vi "neuKLEIN.vi"() -> ()   [LabVIEW 2016] (continued)
  in  "FPGA_DIO_Labels":T54={"Array"=["PB_0.20 - Image Freq Selector", "PB_0.12 - Blue Trap or Image Selector", "PB_0.22 - Blue Cold MOT TTL", "PB_0.17 - Blue Hot MOT Freq Selector", "***** BROKEN ***** BNC snapped, just needs to be replaced", "PB_0.19 - ODT Dimple (Sheet) Light Trigger", "PB_0.21 - ODT Loading Trap Light Trigger", "PB_1.00 - B field - Switch 0", "PB_1.07 - LCR Switch", "PB_1.10 - B field - Switch 1", "", "", "", "", "", "", "", "", "", "", " ", "", "", ""], "PB_0_Ch_Labels\n"=["0", "1", "2", "3", "4", "5", "6", "7", "8", "9", "10", "11", "12", "13", "14", "15", "16", "17", "18", "19", "20", "21", "22", "23", "24", "25", "26", "27", "28", "29", "30", "31"]}
  in  "FPGA_AO_Labels":T54={"Array"=["************BORKED************", "************BORKED************", "Blue MOT B-field gradient (external ADG419 switches to Red MOT gradient)", "6221 (ODT card) Waveform trigger", "X Trim Coil (Driving BioChip)", "Y Trim Coil", "Z Trim Coil", "LCR Setting", "Blue Laser Frequency Selector", "Blue MOT Power Setpoint", "", "", "", "", "", "", "", "", "", "", " ", "", "", ""], "PB_0_Ch_Labels\n"=["0", "1", "2", "3", "4", "5", "6", "7", "8", "9", "10", "11", "12", "13", "14", "15", "16", "17", "18", "19", "20", "21", "22", "23"]}
  in  "Update FPGA Ctrl":bool
  out "get_loop_time":u32
  out "error out":errorcluster={"status"=TRUE, "code"=-2145378293, "source"="Initboard.vi: Unknown or reserved error"}
  out "Handle Out":i16=16384
  out "Pico Scope Info":T55={"Driver Version"="1.1.4.20", "USB Version"="2.0", "Hardware"="1", "Variant"="5243B", "Batch and Serial"="CW334/117", "Cal Date"="20Mar14", "Kernel Version"="1.0", "Digital HW Version"="1", "Analogue HW Version"="1", "Firmware 1"="1.3.3.0", "Firmware 2"="1.0.24.0"}
  out "Control Reference Cluster":T56={"Controls[]"=[refnum, refnum, refnum, refnum, refnum, refnum, refnum, refnum, refnum, refnum, refnum, refnum, refnum, refnum, refnum, refnum, refnum, refnum, refnum, refnum, refnum, refnum, refnum, refnum, refnum, refnum, refnum, refnum, refnum, refnum, refnum, refnum, refnum, refnum, refnum, refnum, refnum, refnum, refnum, refnum, refnum, refnum, refnum, refnum, refnum, refnum, refnum, refnum, refnum, refnum, refnum, refnum, refnum, refnum, refnum, refnum, refnum, refnum, refnum, refnum, refnum, refnum, refnum, refnum, refnum, refnum, refnum, refnum, refnum, refnum, refnum, refnum, refnum, refnum, refnum, refnum, refnum, refnum, refnum, refnum, refnum, refnum, refnum, refnum, refnum, refnum], "Control Names"=["Control Tab Control", "Start Experiment", "Shutdown Experiment", "Exp Running", "Camera Ready", "Trigger Snap Mode", "Number", "Set Analysis Mode", "Temp. (K) - X", "Temp. (K) - Y", "Drop Time", "Scan Name", "Current Param. Values", "output cluster", "Take Pictures", "Abort Scan", "Scan Progress", "Information Tab Control", "Trap Frequencies", "Phase Space Density", "Break Loop", "Picoscope Ready", "Wavemeter", "Stat. Limits", "Num and Temp Stats", "Stats Flag", "cRIO Ready", "XML File Location", "Load", "XML Filename", "SaveButton", "current spinal_column MD5", "Agilent E3631A Settings", "Program Agilent", "PicoScope", "Intitialize PicoScope", "Novatech Synth Settings", "Synth Notes", "FPGA_panel_tab_ctrl", "6229 Green Lattice Inputs", "Green Lattice Waveform Graph", "ODT Params", "ODT Waveform Graph", "Red MOT 87 Inputs", "Red 87 Waveform Graph", "Red MOT 87 Notes", "Red MOT 88 Inputs", "Red 88 Waveform Graph", "Red MOT 88 Notes", "6713 Blue MOT", "Blue MOT Waveform Graph", "Blue MOT Trapping Notes", "PixelFly Status", "Buffer status", "PixelFly Controls", "Experimental Variables", "Calculated Experimental Values", "Scan Parameters", "48ch_pb_array", "PB_Labels_Tab", "error out", "Pico Scope Info", "Handle Out", "Control Reference Cluster", "Update FPGA Ctrl", "FPGA_AO_Labels", "FPGA_DIO_Labels", "get_loop_time", "GIANT Atoms", "Giant Data Cuts", "Pico Scope Channel A", "Pico Scope Channel B", "Atom Image", "Background Image", "Atoms - BG", "Atom Closeup", "OD", "Atom Number Chart", "Data Cuts", "Best Fit Parameter Cluster", "Elapsed time ( ms)", "Temperature Chart", "FPGA_Labels", "FPGA_cntrl", "pb_label_cluster 2", "pb_label_cluster"]}
  # "Select a PB Channel to set with a phase time for evaporation or whatever"
  # "Camera Controls"
  # "Camera Indicators"
  # "NOTE: 2015.10.19 - Jim\nDouble Shot is currently the only image mode supported.\nBackground subtraction will fail if the mode is changed"
  # "Status flags"
  # "Buffer errors"
  # "Memory usage"
  # "Center Freq. [MHz] (0)"
  # "Dither Amp. [kHz] (1)"
  # "Red Boson Power (2)"
  # "Red B-Field Gradient (3)"
  # "OUTPUT UNRELIABLE (4)"
  # "Image VCO Freq. (5)"
  # "Blue MOT VCO Freq. (6)"
  # "Spin Pol VCA (7)"
  # "Trap - Center Freq. (0)"
  # "Trap - Dither Amp. (1)"
  # "Trap - Power (2)"
  # "Z Trim [LO] (3)"
  # "Stir - Center Freq. (4)"
  # "Stir - Dither Amp. (5)"
  # "Stir - Power (6)"
  # "Z Trim [HI] (7)"
  # "Notes below cluster describe the variables used for each formula and \neach variable has a designation of SET or CALC as explained here\n\nSET - user defined, defines the output waveform \nCALC - program calculated value that will be updated in the entry field, input is ignored"
  # "Difference between \"Evaporation Formula\" and \"Evap - Calc Tau\" is mostly in defining\nthe endpoint of the trajectory. By calculating tau you can specify the final voltage of\nthe waveform."
  # "Power Law\ny = const + (init - const)* t^eta\n\nConstant - SET - constant offset\nInitial Value - SET - starting point for ramp\nFinal Value - CALC - final value of waveform at the end of the phase\nTau - CALC - forced to zero (not used for power law)\nEta - SET - power law dependence on time, positive (neg causes error)"
  # "Evaporation Formula\ny = const +  (init - const) / (1 + t/tau)^beta\nbeta is a function of eta as defined in PRA 64, 051403 \n\nConstant - SET - constant offset\nInitial Value - SET - starting point for ramp\nFinal Value - CALC - final value of waveform at the end of the phase\nTau - SET - time constant for the evaporation\nEta - SET - ratio of temperature over trap depth"
  # "Evap - Calc Tau\ny =  init / (1 + t/tau)^beta\ntau =  tf * (1 / ( 1 - ( final / init ))**(1 / beta) - 1)\ntf is the final time (total phase time)\nbeta is a function of eta\n\nConstant - CALC - forced to zero (not used)\nInitial Value - SET - starting point for ramp\nFinal Value - SET - final value of waveform at the end of the phase\nTau - CALC - time constant for the evaporation\nEta - SET - ratio of temperature over trap depth"
  # "Notes below  describe the variables used for each formula and each variable has a designation of SET or NA as explained here\n\nSET - user defined, defines the output waveform \nNA - input in this field is ignored for this function\n\nConversion selection is currently disabled (2018.11.01) can be enabled by modifying the Arb Waveform subvi to include calc"
  # "Evap - Calc Tau\ny =  init / (1 + t/tau)^beta\ntau =  tf * (1 / ( 1 - ( final / init ))**(1 / beta) - 1)\ntf is the final time (total phase time)\nbeta is a function of eta\n\nConstant - CALC - forced to zero (not used)\nInitial Value - SET - starting point for ramp\nFinal Value - SET - final value of waveform at \n                                 the end of the phase\nTau - CALC - time constant for the evaporation\nEta - SET - ratio of temperature over trap depth"
  # "Power Law\ny = const + (init - const)* t^eta\n\nConstant - SET - constant offset\nInitial Value - SET - starting point for ramp\nFinal Value - SET - final value of waveform at the end of the phase\nTau - CALC - forced to zero (not used for power law)\nEta - SET - power law dependence on time, positive (neg causes error)"
  # "Exponential\ny = (vo-constant) * exp(t/(tau)) + constant;\ntau = time / ln(vf/(vo-constant)); (time is the total phase time)\n\nConstant - SET - constant offset\nInitial Value - SET - starting point for ramp\nFinal Value - SET - final value of waveform at the end of the phase)\nDegree - NA"
  # "Evaporation Formula\ny = const +  (init - const) / (1 + t/tau)^beta\nbeta is a function of eta as defined in PRA 64, 051403 \n\nConstant - SET - constant offset\nInitial Value - SET - starting point for ramp\nFinal Value - CALC - final value of waveform at \n                                     the end of the phase\nTau - SET - time constant for the evaporation\nEta - SET - ratio of temperature over trap depth"
  # "Constant\ny = Constant + Initial + Final; \n\nConstant - SET - can still be used for conversions - constant offset\nInitial Value - SET - starting point for ramp\nFinal Value - SET\nDegree - NA"
  # "Tanh\ny = (vf - vo)/2*(tanh(slope*2*pi*t - slope*pi) +1) + vo; \n\nConstant - NA - can still be used for conversions - constant offset\nInitial Value - SET - starting point for ramp\nFinal Value - SET - Final value of the ramp\nDegree - SET - sets the slope of the Tanh (bigger is steeper)"
  # "Difference between \"Evaporation Formula\" and \"Evap - Calc Tau\" is mostly in defining\nthe endpoint of the trajectory. By calculating tau you can specify the final voltage of\nthe waveform."
  # "(0) Arm A"
  # "(1) Arm B"
  # "(2) Arm C"
  # "(3) Unused"
  # "(0) Arm A"
  # "(1) Arm B"
  # "(2) Arm C"
  # "(3) Unused"
  # "Constant Operation Control"
  # "Boolean Operation Control"
  # "Custom Operation Controls"
  # "Constant Operation Control"
  # "Boolean Operation Control"
  # "Custom Operation Controls"
  # "Constant Operation Control"
  # "Boolean Operation Control"
  # "Custom Operation Controls"
  # "Constant Operation Control"
  # "Boolean Operation Control"
  # "Custom Operation Controls"
  # "Constant Operation Control"
  # "Boolean Operation Control"
  # "Custom Operation Controls"
  # "Constant Operation Control"
  # "Boolean Operation Control"
  # "Custom Operation Controls"
  # "Constant Operation Control"
  # "Boolean Operation Control"
  # "Custom Operation Controls"
  # "Constant Operation Control"
  # "Boolean Operation Control"
  # "Custom Operation Controls"
  # "Constant Operation Control"
  # "Boolean Operation Control"
  # "Custom Operation Controls"
  # "Constant Operation Control"
  # "Boolean Operation Control"
  # "Custom Operation Controls"
  # "Constant Operation Control"
  # "Boolean Operation Control"
  # "Custom Operation Controls"
  # "Constant Operation Control"
  # "Boolean Operation Control"
  # "Custom Operation Controls"
  # "Constant Operation Control"
  # "Boolean Operation Control"
  # "Custom Operation Controls"
  # "Constant Operation Control"
  # "Boolean Operation Control"
  # "Custom Operation Controls"
  # "Constant Operation Control"
  # "Boolean Operation Control"
  # "Custom Operation Controls"
  # "Constant Operation Control"
  # "Boolean Operation Control"
  # "Custom Operation Controls"
  # "Synth Layout\n---------------------\nSyn. 0   |   Syn. 1   | \n-------- |---------- |\nSyn. 2   |   Syn. 3   |\n\n*2D grid is collapsed to 1D so be careful with addressing if adding more synths"
  # "Things to do for Pico VI\n2017.09.11 \n- Make this control more versatile, not only having the conversions work at 15bit resolution and the threshold needs to work for any range setting\n- Auto trigger time should have option to set time to wait as some factor of the total experimental time (like 1.2*(total PB time)"
  # "2016.12.12 - Currently back-end cnoversion assume the scope is in 15bit mode with the range at 5V."
  # "2018.10.31\nNOTE: (JAA) This triggerable functionality of the Agilent has been abandoned. It kind of works but is not reliable. The code should be taken out of the program entirely and only the single-use programmable piece should be kept (the part activated by pressing Program Agilent) as this is the reliable bit of code."
  # "Since the Agilent is slow to communicate the program will skip programming if the \"Auto Program Agilent\" switch is disabled.  If \"Auto Program\" is enabled the settings to the far left are used to program the Agilent.\n\nAdditionally, the Agilent has an internal software trigger that can a single channel between two current setpoints. The clock is not referenced to the Pulseblaster so be careful with timing when using the Triggered Agilent Settings. To enabled this mode use the \"Agilent Software Trigger\" swithc.\n\nUse the \"Program Agilent\" button to perform a one-time write (with settings on the far left) to avoid having the slow response of the supply during data scans.\n\nNOTE: When setting only current values the program will default to setting the maximum allowed voltage for a given channel."
  # "6V (2017.06.15)\n\nReported Current = \nSet Cur - 0.003A\n\nActual Current = \nSet Cur - 0.0015A"
  # "+25V (2017.06.15)\n\nReported Current = \nSet Cur + 0.002A\n\nActual Current = \nSet Cur + 0.002A"
  # "-25V (2017.06.15)\n\nReported Current = \nSet Cur\n\nActual Current = \nSet Cur"
  # "Beware of the offset in set, reported and actual current from Agilent channels. Below are corrections measured for each channel"
  # "--25V  Measurements"
  # "+25V  Measurements"
  # "6V  Measurements"
  # "-25V Output Settings"
  # "+25V Output Settings"
  # "6V Output Settings"
  # "When saving and loading the .dat file for experiments, you must ensure that the type definition is consistent between the version of spinal_column you are attempting to use. (i.e. the saved data type def and the current version type def must be exactly the same)\n\nThe MD5 hash is a unique string for the current status of the spinal column type defintiion. This MD5 will be saved into the filename for the dat files and checked when loading files."
  # "Click to save an xml file of the current experimental parameters\nto the raw_data folder indicated in the \"scan parameters\" tab"
  # "of"
  # "<-- Pump Side"
  # "Source Side -->"
  # "Digital Input Labels"
  # "IMPORTANT INFO:\n\n- For explanations of the available operations please refer to the \"FPGA operations.pdf\" file included in the neuKLEIN project.\n(In manual describe how you have to deploy the library to the RT target. Really need to get references for learning)\n\n- When using the scan functionality to take data, Channel to change will identify the channel while Phase to change will only be used for the \"Custom operation\" where it identifies which Output Value to change. The constant & Boolean operations have separate cases for controllnig these outputs.\n\n- BOP protection causes jumps greater than 1.5A to be ramped at a rate of 100A/s (or 100mA/ms). When the current gets within 1.5A the control voltage will jump the BOP to the final setpoint."
  # "Analog Output Labels"
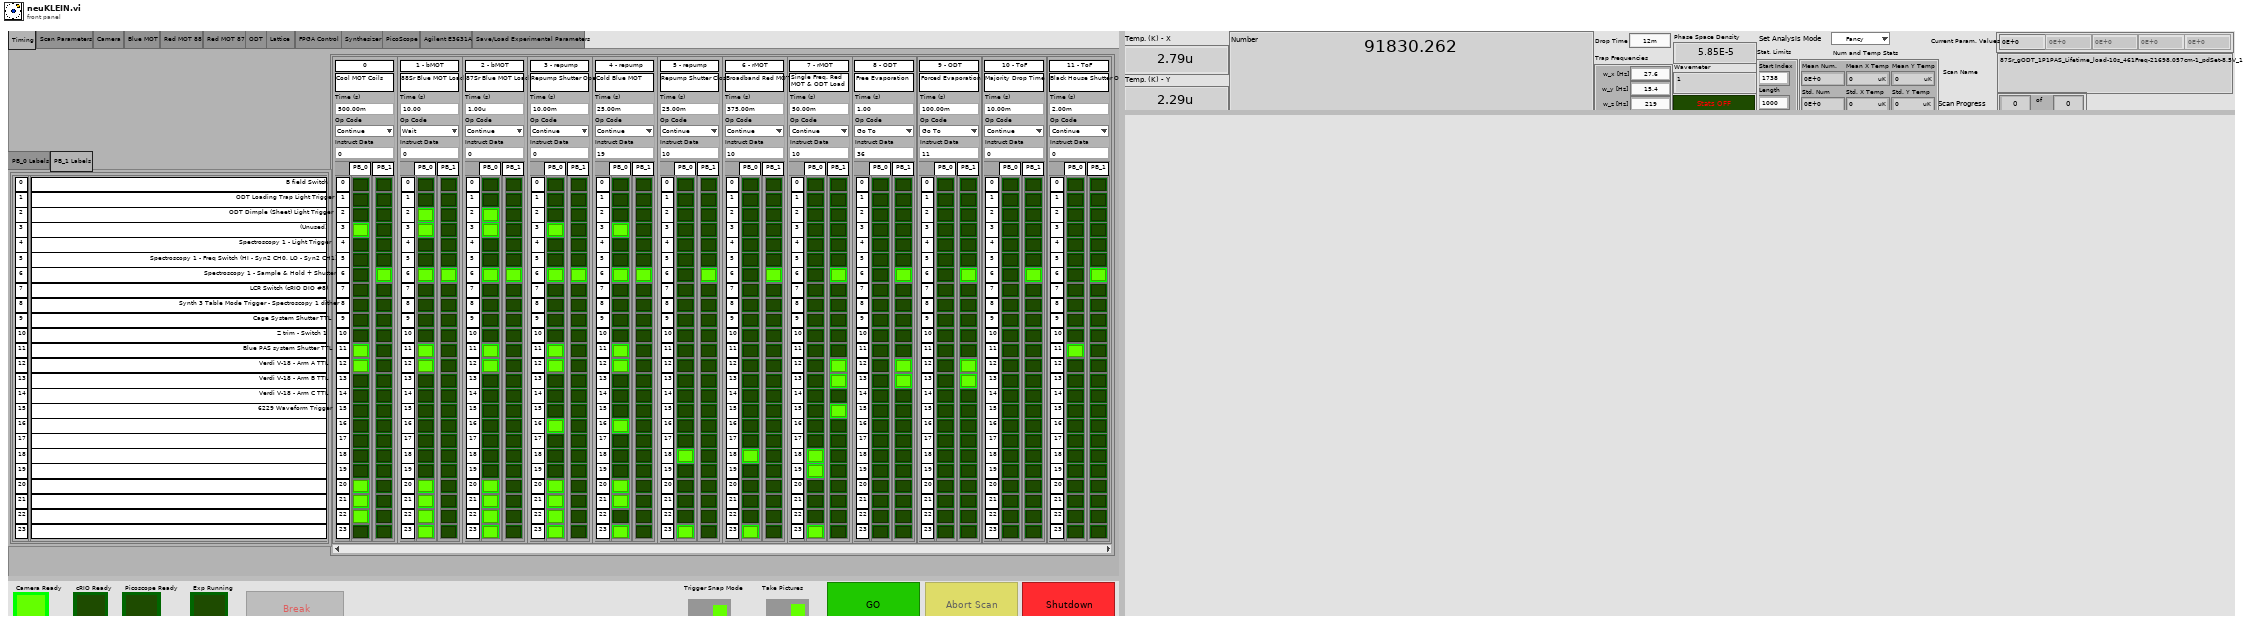
[diagram p1: front panel]
types:
  T1 = enum32{"Timing", "Scan Parameters", "Camera", "Blue MOT", "Red MOT 88", "Red MOT 87", "ODT", "Lattice", "FPGA Control", "Synthesizer", "PicoScope", "Agilent E3631A", "Save/Load Experimental Parameters"}
  T2 = typedef "pb_labels_v2.ctl" = cluster{"Array":string[], "PB_0_Ch_Labels\n":string[]}
  T3 = typedef "48ch_pb_array.ctl" = T4[]
  T4 = typedef "48ch_single_timing_column_condensed.ctl" = cluster{"Label and Instructions":cluster{"Column Number":string, "Comments":string, "Time (s)        ":dbl, "Op Code":i32, "Instruct Data":i32}, "PB_1_Bools":bool[], "Column Number":string, "Column Number 2":string, "PB_0_Bools":bool[], "Ch_Labels":string[]}
  T5 = typedef "ScanParametersPanel.ctl" = cluster{"Initial Values":dbl[], "Final Values":dbl[], "Step Sizes":dbl[], "Parameters to Change":T6[], "Channels to Change":u32[], "Number of Parameters to Scan":i32, "Parameter Nickname (no spaces)":string[], "Scan Base Name":string, "Raw_Data Folder":path, "ROI Parameters":T7, "Drop Time (ms)":dbl, "Phases To Change":u32[], "Scan Pulseblaster Channel With Parameter":T8, "Preserve Waveform\nContinuity":bool, "Generated Array Type":enum16{"Custom Array From File", "Default (old way)"}, "Master Batch Third Column":dbl, "Master Batch Fourth Column":dbl, "Master Batch Fifth Column":dbl, "Current Param. Values":dbl[]}
  T6 = typedef "ParameterToChange.ctl" = enum16{"Dummy Variable", "Synth Amplitude", "Synth Frequency", "Synth Phase", "ODT Params Phase Time", "ODT Params Tau", "ODT Params Final Voltage", "ODT Params Initial Voltage", "ODT Params Eta", "Red Mot 88 Phase Time", "Red Mot 87 Phase Time", "Red Mot 88 Final Voltage", "Red Mot 88 Initial Voltage", "Red Mot 87 Final Voltage", "Red Mot 87 Initial Voltage", "PulseBlaster", "6713 Voltage", "Green Lattice Phase Time", "Green Lattice Initial Voltage", "Green Lattice Final Voltage", "Agilent Current Setpoint", "FPGA - Constant Op - Set", "FPGA - Bool Op - Output HI", "FPGA - Bool Op - Output LO", "FPGA - Custom Op"}
  T7 = typedef "ROI_set.ctl" = cluster{"Background Radius":dbl, "Atom Radius":dbl, "X Center":dbl, "Y Center":dbl}
  T8 = typedef "ScanPBandParam.ctl" = cluster{"Change PB Time Toggle":bool, "PB Channel":dbl, "Parameter Number":dbl}
  T9 = typedef "experimentalvariables.ctl" = cluster{"Pixel Size before binning (µm)":dbl, "Imaging Wavelength (m)":dbl, "Isotope":i32, "1P1 Linewidth (MHz)":dbl, "Imaging Detuning (MHz)":dbl, "Software Bin Size":u16, "Exp. Trigger ON time (ms)":dbl, "Path to spinapi.dll":path, "PB clock_freq (MHz)":dbl}
  T10 = cluster{"Absorption Cross Section (µm)":dbl, "Effective Pixel Area (µm^2)":dbl, "Effective Pixel Size (µm)":dbl}
  T11 = typedef "PixelFly_Control.ctl" = cluster{"Acquitsition Settings":T12, "Initialization":cluster{"Exposure mode":u16, "exp time":i32, "exp level":i32, "gain":i32, "boardid in":i32, "offset":i32, "V bin":i32, "H bin":i32, "trigger":bool, "Bit depth":T13}}
  T12 = typedef "Acquisition Settings.ctl" = cluster{"Buffer number":i32, "Size (Bytes)":i32, "initialized array":u16[][], "X Bin":i32, "Y Bin":i32, "Board Handle":u32, "Picture parameters":cluster{"ccdxsize":i32, "ccdy":i32, "pictx":i32, "picty":i32, "bitspixel":i32}, "Buffer Out":u16[]}
  T13 = typedef "Bit_Depth_Enum.ctl" = i32
  T14 = typedef "PixelFly Buffer Status.ctl" = cluster{"Write":bool, "Write done":bool, "Queued":bool, "Cancelled":bool, "Select":bool, "Select done":bool, "Burst":bool, "Size":bool, "Event":bool, "Timeout":bool, "Open":i32, "Map":i32, "Exposure":i32[], "Offset":i32[], "Size":i32[], "Transfer":i32[], "Total Size":i32}
  T15 = typedef "PixelFly Status Indicator.ctl" = cluster{"Board Parameters":cluster{"Type":u32, "Number":u32, "Initialized":bool, "Running":bool, "Lost head":bool, "CCD X size":u32, "CCD Y size":u32, "Mode":u32, "Exposure time":u32, "Exposure level":u32, "Horizontal bin":u32, "Vertical bin":u32, "Reg W":bool, "Gain":u32, "Pixel depth":i32, "Bit Shift":u32, "Offset":u32, "Last exposure":u32, "Double ":bool, "Light meter":bool, "Color":bool, "Open count":u32, "Active buffer":bool, "Next Buffer":bool}, "CCD temp":i32}
  T16 = typedef "6713_waveform_generation.ctl" = cluster{"Active Device":string, "Active Channels":bool[], "Waveform Parameters":T17, "Active Phases":bool[], "Phase Times":dbl[], "Trigger Channel":tag, "FIFO Buffer Size":dbl, "6713_ch_labels":T20}
  T17 = typedef "6713_waveform_parameter_array.ctl" = T18[][]
  T18 = typedef "6713_static_waveform_item.ctl" = cluster{"Constant":dbl, "Nickname":string, "Conversion":T19}
  T19 = typedef "Neutral_voltage_conversion_control.ctl" = enum16{"Volts", "B Field Grad (G/cm)", "Red Boson Cntr Freq (MHz)", "Red Boson Dither Amp (kHz)", "Red Boson Power (mW)", "Red 87 Trap Cntr Freq (MHz)", "Red 87 Trap Dither Amp (kHz)", "Red 87 Trap Power (mW)", "Red 87 Stir Cntr Freq (MHz)", "Red 87 Stir Dither Amp (kHz)", "Red 87 Stir Power (mW)", "ODT Sheet Trap Power (W)", "ODT Loading Trap Power (W)"}
  T20 = typedef "6713_ch_labels.ctl" = cluster{"Array":string[], "PB_0_Ch_Labels\n":string[]}
  T21 = typedef "6733_control_panel.ctl" = cluster{"Active Device":string, "Active Channels":bool[], "Waveform Parameters":T22, "Active Phases":bool[], "Phase Times":dbl[], "Trigger Channel":T24}
  T22 = typedef "6733_waveform_parameter_array.ctl" = T23[][]
  T23 = typedef "6733_waveform_item.ctl" = cluster{"Function":enum16{"Polynomial", "Exponential", "Constant", "Tanh"}, "Initial":dbl, "Final":dbl, "Degree":dbl, "Nickname":string, "Conversion":T19, "Constant":dbl}
  T24 = typedef "Trigger_Channel_Selector.ctl" = tag
  T25 = typedef "6221_panel.ctl" = cluster{"Waveform Parameters":T26, "Active Phases":bool[], "Active Channels":bool[], "Phase Times (s)":dbl[], "Active Device":string, "Trigger Channel":tag, "Evaporation Phase":dbl, "Evaporation Channel":dbl}
  T26 = typedef "6221_waveform_input.ctl" = T27[][]
  T27 = typedef "6221_waveform_param.ctl" = cluster{"Initial Value":dbl, "Final Value":dbl, "Tau":dbl, "Eta":dbl, "Nickname":string, "Function Type":enum16{"Constant", "Power Law", "Evap - Calc Tau", "Evaporation Formula", "Tanh", "Exponential"}, "Conversion":T19, "Constant":dbl}
  T28 = typedef "6229_arb_waveform_generation.ctl" = cluster{"Active Device":string, "Active Channels":bool[], "Active Phases":bool[], "Phase Times":dbl[], "Trigger Channel":tag, "FIFO Buffer Size":dbl, "Sample Step Time (us)":dbl, "Initialization Parameters":cluster{"Enable Initialization":bool, "Initial Values":dbl[]}, "Waveform Parameters":T29}
  T29 = typedef "6229_evap_waveform_input.ctl" = T27[][]
  T30 = typedef "op_ctrl_cluster.ctl" = cluster{"Channel 0":T31, "Channel 1":T31, "Channel 2":T31, "Channel 3":T31, "Channel 4":T31, "Channel 5":T31, "Channel 6":T31, "Channel 7":T31, "Channel 8":T31, "Channel 9":T31, "Channel 10":T31, "Channel 11":T31, "Channel 12":T31, "Channel 13":T31, "Channel 14":T31, "Channel 15":T31}
  T31 = typedef "op_ctrl_element.ctl" = cluster{"Operation":i16, "Input A":T32, "Output - LO":T33, "Output - HI":T33, "Inputs":T32[], "Output Values":T33[], "Num. Inputs":i32, "Set Point":T33, "Inv.":bool[], "Inv. A":bool, "Inv. B":bool, "Input B":T32}
  T32 = typedef "DIO_selector.ctl" = i32
  T33 = typedef "output_value.ctl" = fxp<+/-,20,5>
  T34 = typedef "op_label_cluster.ctl" = cluster{"Channel 0":T35, "Channel 1":T35, "Channel 2":T35, "Channel 3":T35, "Channel 4":T35, "Channel 6":T35, "Channel 5":T35, "Channel 7":T35, "Channel 8":T35, "Channel 9":T35, "Channel 10":T35, "Channel 11":T35, "Channel 12":T35, "Channel 13":T35, "Channel 14":T35, "Channel 15":T35}
  T35 = typedef "op_label_element.ctl" = cluster{"Channel Description":string}
  T36 = typedef "Synth_controls.ctl" = cluster{"Channel Settings":T37[], "Active Chans":bool[], "COM Port":refnum<visa-resource-name>, "Table Mode":T38}
  T37 = typedef "synth_channel.ctl" = cluster{"Voltage (Amp.) ":dbl, "Frequency (MHz)":dbl, "Phase (deg)":dbl, "Nickname":string}
  T38 = typedef "table_mode.ctl" = cluster{"Initial Freq.(MHz)":dbl, "FinalFreq":dbl, "Freq. Step (MHz)":dbl, "Voltage (Amp.)":dbl, "Asc. & Desc.":bool, "Custom Frequencies":dbl[], "Custom Amplitude":dbl[], "Table Mode Switch":bool, "Array Gen":enum16{"Auto", "Custom"}, "Randomize":bool, "Continuous":bool}
  T39 = typedef "pico_control_panel.ctl" = cluster{"Channel A Settings":T40, "Channel B Settings":T40, "Trigger Options":T41, "Pico Scope Inititalization Settings":T42, "Use PicoScope?":bool, "Acquisition Settings":cluster{"Pre Trigger Time (s)":dbl, "Post Trigger Time (s)":dbl, "Resolution (s)":dbl, "Four Channel Device":bool, "Number of Captures":dbl}}
  T40 = typedef "pico_channel_settings.ctl" = cluster{"Enabled":bool, "Coupling":i16, "Range":u16, "Analogue Offset":sgl}
  T41 = typedef "pico_trigger.ctl" = cluster{"Trigger Enabled":bool, "Trigger Source":enum16{"Channel A", "Channel B", "Channel C", "Channel D", "Ext."}, "Trigger Threshold (-5 to 5 V)":dbl, "Trigger Slope":u16, "Trigger Delay (s)":dbl, "Auto Trigger Time (ms)":i16}
  T42 = typedef "pico_init_settings.ctl" = cluster{"USB Power":bool, "Use Serial Number":bool, "Resolution":i32, "Serial Number":string, "Handle":i16}
  T43 = typedef "Settings_Control.ctl" = cluster{"VISA resource name":refnum<visa-resource-name>, "Voltage Set (6V max)":dbl, "Current Set (5A max)":dbl, "Voltage Set (25V max)":dbl, "Current Set (1A max)":dbl, "Voltage Set (-25V max)":dbl, "Current Set (1A max)":dbl, "6V Switch":bool, "+25V Switch":bool, "-25V Switch":bool, "Agilent E3631A Measurements":T44, "Triggered Agilent Settings":T45, "Auto Program Agilent":bool, "Agilent Software Trigger":bool}
  T44 = typedef "Measurement_Indicator.ctl" = cluster{"6V Actual Voltage Level (V)":dbl, "6V Actual Current Level (A)":dbl, "25V Actual Voltage Level (V)":dbl, "25V Actual Current Level (A)":dbl, "-25V Actual Current Level (A)":dbl, "-25V Actual Voltage Level (V)":dbl}
  T45 = typedef "Trigger_Settings.ctl" = cluster{"Trigger \nDelay (s)":dbl, "Enable +6V Channel":bool, "+6V Current":dbl, "Enable -25V Channel":bool, "-25V Current":dbl, "Enable +25V Channel":bool, "+25V Current":dbl}
  T46 = typedef "output_cluster.ctl" = cluster{"Number":dbl, "OD":dbl[][], "Data Cuts":dbl[][], "Temperature (K) x":dbl, "Temperature (K) y":dbl}
  T47 = typedef "numAndTempStats.ctl" = cluster{"Mean Num.":dbl, "Std. Num":dbl, "Mean X Temp":dbl, "Std. X Temp":dbl, "Mean Y Temp":dbl, "Std. Y Temp":dbl}
  T48 = cluster{"w_x [Hz]":dbl, "w_y [Hz]":dbl, "w_z [Hz]":dbl}
  T49 = typedef "Progress_Indicator.ctl" = cluster{"Current Pnt Num":i32, "Total Num Pts":i32}
  T50 = enum32{"Standard Image Information", "Picoscope traces", "Large OD Image", "cRIO Information", "Error Information"}
  T51 = cluster{"Temperature (K) x":dbl, "Temperature (K) y":dbl}
  T52 = typedef "Fit Parameter Cluster.ctl" = cluster{"Amplitude (OD)":dbl, "X Center (px)":dbl, "Y Center (px)":dbl, " X Width (um)":dbl, "Y Width (um)":dbl, "Aspect Ratio":dbl, "Rot. Angle (deg)":dbl}
  T53 = cluster{"Channel A Out":dbl[], "Channel A Out":dbl[]}[]
  T54 = typedef "portAssign_labels.ctl" = cluster{"Array":string[], "PB_0_Ch_Labels\n":string[]}
  T55 = cluster{"Driver Version":string, "USB Version":string, "Hardware":string, "Variant":string, "Batch and Serial":string, "Cal Date":string, "Kernel Version":string, "Digital HW Version":string, "Analogue HW Version":string, "Firmware 1":string, "Firmware 2":string}
  T56 = cluster{"Controls[]":refnum<vi>[], "Control Names":string[]}
  T57 = typedef "rydberg_state_machine_states.ctl" = enum16{"Initialize", "Idle", "Experiment Running", "Trigger Snap Mode", "Scan Mode", "Load Experiment", "Shutdown"}
  T58 = enum8{"Enabled", "Disabled", "Disabled and Grayed Out"}
  T59 = cluster{"Experimental Variables":T9, "Red MOT 88 Inputs":T21, "6713 Blue MOT":T16, "48ch_pb_array":T3, "Red MOT 87 Inputs":T21, "ODT Params":T25, "Agilent E3631A Settings":T43, "PixelFly Controls":T11, "Scan Parameters":T5, "PicoScope":T39, "6229 Green Lattice Inputs":T28, "Novatech Synth Settings":T36[][], "Control Reference Cluster":cluster{"Controls[]":refnum<vi>[], "Control Names":string[]}, "FPGA_cntrl":T30}
  T60 = cluster{"Initial Values":refnum<vi>, "Final Values":refnum<vi>, "Step Sizes":refnum<vi>}
  T61 = cluster{"Channels to Change":refnum<vi>, "Phases To Change":refnum<vi>}
  T62 = typedef "DialogType.ctl" = u16
  T63 = typedef "spinal_column.ctl" = cluster{"Experimental Variables":T9, "Red MOT 88 Inputs":T21, "6713 Blue MOT":T16, "48ch_pb_array":T3, "Red MOT 87 Inputs":T21, "ODT Params":T25, "Agilent E3631A Settings":T43, "PixelFly Controls":T11, "Scan Parameters":T5, "PicoScope":T39, "6229 Green Lattice Inputs":T28, "Novatech Synth Settings":T36[][], "Control Reference Cluster":cluster{"Controls[]":refnum<vi>[], "Control Names":string[]}, "FPGA_cntrl":T30}
  T64 = typedef "LVCursorListTypeDef.ctl" = cluster{"Name":string, "Color":u32, "Style":u8, "Point Style":u8, "Name Visible":bool, "Allow Drag":bool, "Cursor Mode":u32, "Plot":i32, "Index":i32, "Position":cluster{"X":dbl, "Y":dbl}, "X Scale":u32, "Y Scale":u32, "Watch Plots":i32[], "Watch All Plots":bool, "Plot Area":i32, "Label Offset":cluster{"X":dbl, "Y":dbl}}[]
  T65 = cluster{"Temperature (K) x":dbl, "Temperature (K) y":dbl}[]
  T66 = cluster{"XScale.Maximum":dbl, "History Data":dbl[], "History Data":cluster{"Temperature (K) x":dbl, "Temperature (K) y":dbl}[]}
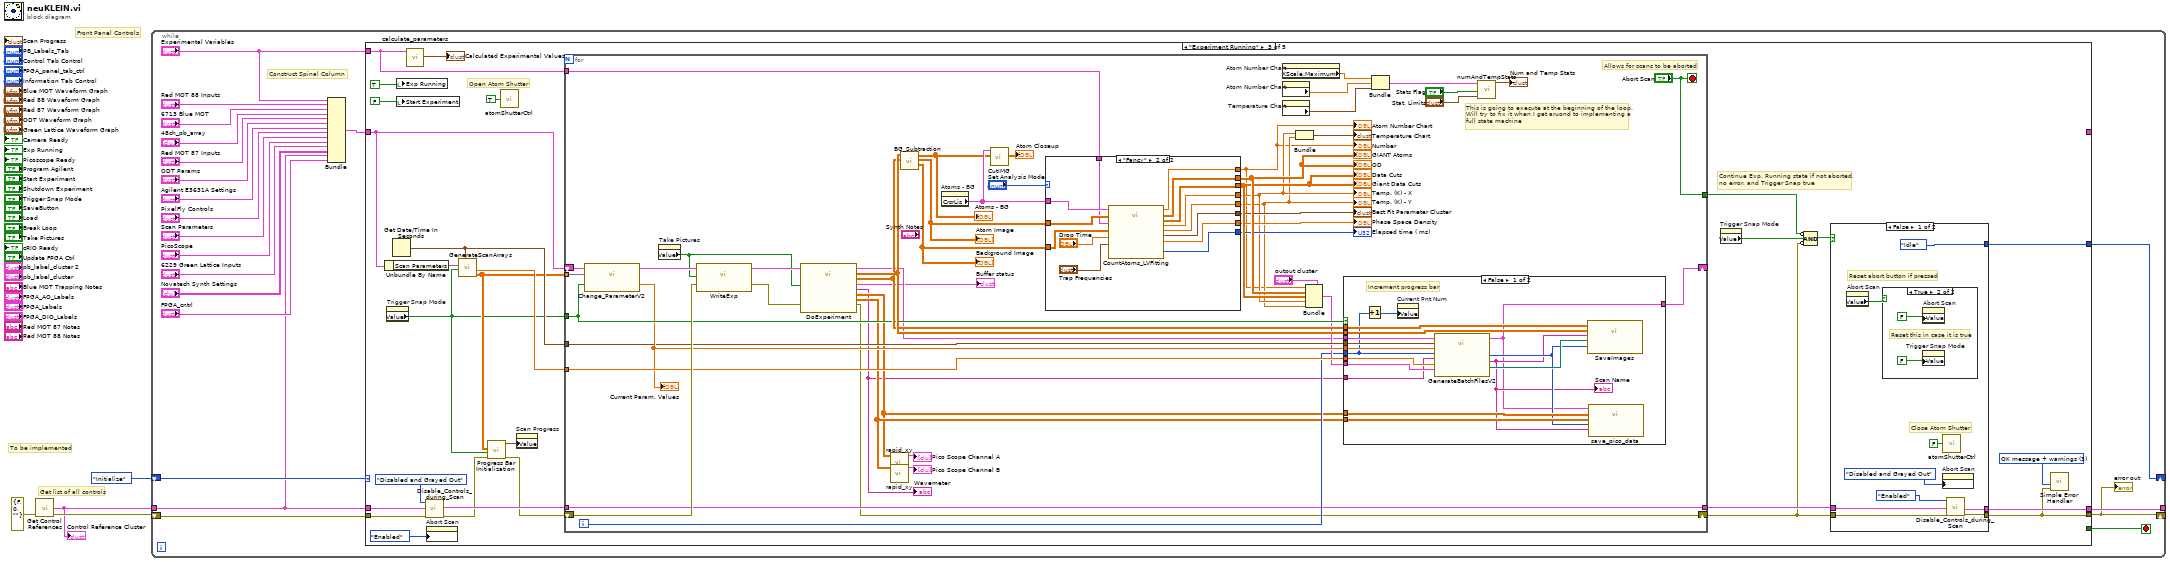
[diagram p0: block diagram]
diagram:
  # "To be implemented"
  # "Get list of all controls"
  # "Front Panel Controls"
  n1 = call "Get Control References.vi"("error in"=errorcluster {"status"=FALSE, "code"=0, "source"=""} ("error constant")) -> ("error out"=w2:errorcluster, "Control Reference Cluster"=w1:T56)  [unwired: 3 in]
  "Control Reference Cluster" <- w1
  n2 = while {
    shift-right: [w23] -> _
    shift-left: rydberg_state_machine_states."Initialize" -> [w25]
    shift-right: [w7] -> _
    shift-left: w2 -> [w24]
    tunnel: w1 -> [w5]
    tunnel: [w12] -> _
    stop <- w22 stop-if-true
    # "Construct Spinal Column"
    n3 = Bundle("Experimental Variables"="Experimental Variables", "Red MOT 88 Inputs"="Red MOT 88 Inputs", "6713 Blue MOT"="6713 Blue MOT", "48ch_pb_array"="48ch_pb_array", "Red MOT 87 Inputs"="Red MOT 87 Inputs", "ODT Params"="ODT Params", "Agilent E3631A Settings"="Agilent E3631A Settings", "PixelFly Controls"="PixelFly Controls", "Scan Parameters"="Scan Parameters", "PicoScope"="PicoScope", "6229 Green Lattice Inputs"="6229 Green Lattice Inputs", "Novatech Synth Settings"="Novatech Synth Settings", "Control Reference Cluster"=w5, "FPGA_cntrl"="FPGA_cntrl") -> (w20:T59)  [unwired: 1 in]
    n4 = case shown="\"Experiment Running\"" w25 {
      tunnel: w24 -> [w42 w62 w203 w323 w344]
      tunnel: [w35 w58 w181 w322 w351] -> w7
      tunnel: [rydberg_state_machine_states."Idle" w60 w207 rydberg_state_machine_states."Idle" _] -> w23
      tunnel: [_ w59 _ _ TRUE] -> w22
      tunnel: [_ w57 _ _ w348] -> _
      tunnel: w20 -> [w26 w56 w188 w316 w348]
      tunnel: "Experimental Variables" -> [_ _ w196 _ _]
      tunnel: w5 -> [w37 w55 w191 w326 w350]
      tunnel: [w36 w54 w199 w326 w350] -> w12
      frame "Initialize", Default {
        w34 = T58."Disabled and Grayed Out" ("Disabled")
        w39 = TRUE ("X Scale.Flipped")
        # "Get status of RT app on the cRIO"
        # "Initialize and write value of handle into the picoscope settings"
        # "Set Atom graphs to invert axes so the picture looks correct"
        n5 = Unbundle By Name(w26) -> ("PixelFly Controls"=w32:T11)
        n6 = call "get_spnial_column_MD5.vi"("spinal_column"=w26) -> ("current spinal_column MD5"=→"current spinal_column MD5":string)  [unwired: 10 in]
        n7 = call "pixelfly_init.vi"("error in (no error)"=w42, "PixelFly Controls"=w32) -> ("error out"=w41:errorcluster, "PixelFly Status"=→"PixelFly Status":T15, "PixelFly Controls Out"=w31:T11)  [unwired: 1 in]
        n8 = property on="PixelFly Controls" class="Clust (strict)"("Value"=w31) -> ()  [unwired: 2 in, 2 out]
        n9 = case shown="False" "Intitialize PicoScope" {
          selector: "Intitialize PicoScope" -> [_ w46]
          tunnel: w41 -> [w44 w50]
          tunnel: w26 -> [_ w49]
          tunnel: [w44 w45] -> w30
          frame False {
          }
          frame True {
            n10 = Unbundle By Name(w49) -> ("PicoScope"=w53:T39)
            n11 = property on="Picoscope Ready" class="Bool (strict)"("Value"=TRUE ("Picoscope Ready")) -> ()  [unwired: 2 in, 2 out]
            n12 = call "pico_init.vi"("error in (no error)"=w50, "Initialize PicoScope?"=w46, "PicoScope Acquisition Settings Input"=w53) -> ("error out"=w45:errorcluster, "Unit Info"=→"Pico Scope Info":T55, "Handle Out"=→"Handle Out":i16, "PicoScope Acquisition Settings Output"=w48:T39)  [unwired: 4 in]
            n13 = property on="PicoScope" class="Clust (strict)"("Value"=w48) -> ()  [unwired: 2 in, 2 out]
          }
        }
        n14 = shared-variable "NI-cRIO-9063-01c84dbf\\multiFunc-Lib.lvlib\\rt_app_status"(error in=w30) -> (w28:bool, error out=w29:errorcluster)
        n15 = property on="cRIO Ready" class="Bool (strict)"("Value"=w28) -> ()  [unwired: 2 in, 2 out]
        n16 = property on="Break Loop" class="Bool (strict)"("DisabledEnum"=w34) -> ()  [unwired: 2 in, 2 out]
        n17 = property on="Abort Scan" class="Bool (strict)"("DisabledEnum"=w34) -> ()  [unwired: 2 in, 2 out]
        n18 = property on="Atom Image" class="IntGraph (strict)"("XScale.Flipped"=w39) -> ()  [unwired: 2 in, 2 out]
        n19 = property on="Atom Image" class="IntGraph (strict)"("YScale.Flipped"=w39) -> ()  [unwired: 2 in, 2 out]
        n20 = property on="Atom Closeup" class="IntGraph (strict)"("XScale.Flipped"=w39) -> ()  [unwired: 2 in, 2 out]
        n21 = property on="Atom Closeup" class="IntGraph (strict)"("YScale.Flipped"=w39) -> ()  [unwired: 2 in, 2 out]
        n22 = property on="Atoms - BG" class="IntGraph (strict)"("XScale.Flipped"=w39) -> ()  [unwired: 2 in, 2 out]
        n23 = property on="Atoms - BG" class="IntGraph (strict)"("YScale.Flipped"=w39) -> ()  [unwired: 2 in, 2 out]
        n24 = property on="Background Image" class="IntGraph (strict)"("XScale.Flipped"=w39) -> ()  [unwired: 2 in, 2 out]
        n25 = property on="Background Image" class="IntGraph (strict)"("YScale.Flipped"=w39) -> ()  [unwired: 2 in, 2 out]
        n26 = property on="OD" class="IntGraph (strict)"("XScale.Flipped"=w39) -> ()  [unwired: 2 in, 2 out]
        n27 = property on="OD" class="IntGraph (strict)"("YScale.Flipped"=w39) -> ()  [unwired: 2 in, 2 out]
        n28 = call "Disable_Controls_during_Scan.vi"("Error In"=w29, "Control Reference Cluster Input"=w37, "Control State In"=T58."Enabled" ("Disabled")) -> ("error out"=w35:errorcluster, "Control Reference Cluster Output"=w36:T56)  [unwired: 7 in]
      }
      frame "Idle" {
        n29 = event shown="[4] \"SaveButton\": Value Change" {
          selector: _ -> [_ _ _ _ _ _ _ _]
          dyn-events: _ -> [_ _ _ _ _ _ _ _]
          timeout: 100 -> [_ _ _ _ _ _ _ _]
          tunnel: w62 -> [w83 w105 w119 w135 w149 _ _ _]
          tunnel: [w67 rydberg_state_machine_states."Idle" rydberg_state_machine_states."Idle" rydberg_state_machine_states."Idle" rydberg_state_machine_states."Idle" w162 w168 w176] -> w60
          tunnel: [FALSE _ _ _ _ _ _ _] -> w59
          tunnel: [w66 w104 w118 w134 w148 _ _ _] -> w58
          tunnel: [w77 w106 _ w137 _ _ w167 w175] -> w57
          tunnel: w56 -> [w77 w106 _ w137 w151 _ w167 w175]
          tunnel: w55 -> [w80 _ _ _ _ _ _ _]
          tunnel: [w80 _ _ _ _ _ _ _] -> w54
          event Timeout {
            # "Check if RT app is running"
            # "Change number of scan parameters (could probably be replaced by XControl)"
            # "In case an error is thrown. \nThe program can be shutdown gracefully"
            # "Poll camera for status updates"
            n30 = event-data() -> ()  [unwired: 1 in, 3 out]
            n31 = property on="Shutdown Experiment" class="Bool (strict)"("DisabledEnum"=T58."Enabled" ("Disabled")) -> ()  [unwired: 2 in, 2 out]
            n32 = property on="Exp Running" class="Bool (strict)"("Value"=FALSE ("Exp Running")) -> ()  [unwired: 2 in, 2 out]
            n33 = Unbundle By Name(w77) -> ("Scan Parameters.Number of Parameters to Scan"=w70:i32, "PixelFly Controls.Acquitsition Settings"=w78:T12)
            n34 = property on="PixelFly Status" class="Clust (strict)"() -> ("Value"=w85:T15)  [unwired: 2 in, 2 out]
            n35 = control-ref of="Initial Values"() -> (w90:refnum<vi>)
            n36 = control-ref of="Final Values"() -> (w89:refnum<vi>)
            n37 = control-ref of="Step Sizes"() -> (w88:refnum<vi>)
            n38 = control-ref of="Parameter Nickname (no spaces)"() -> (w86:refnum<vi>)
            n39 = control-ref of="Phases To Change"() -> (w72:refnum<vi>)
            n40 = control-ref of="Parameters to Change"() -> (w71:refnum<vi>)
            n41 = control-ref of="Channels to Change"() -> (w73:refnum<vi>)
            n42 = call "pixelfly_update_status.vi"("error in (no error)"=w83, "PixelFly Status Input"=w85, "Acquitsition Settings"=w78) -> ("error out"=w82:errorcluster, "PixelFly Status Output"=w84:T15)  [unwired: 7 in]
            n43 = Unbundle By Name(w84) -> ("Board Parameters.Initialized"=w81:bool)
            n44 = property on="PixelFly Status" class="Clust (strict)"("Value"=w84) -> ()  [unwired: 2 in, 2 out]
            n45 = Bundle("Initial Values"=w90, "Final Values"=w89, "Step Sizes"=w88) -> (w76:T60)  [unwired: 1 in]
            n46 = Bundle("Channels to Change"=w73, "Phases To Change"=w72) -> (w74:T61)  [unwired: 1 in]
            n47 = Cluster To Array(cluster=w76) -> (array=w87:refnum<vi>[])
            n48 = Cluster To Array(cluster=w74) -> (array=w75:refnum<vi>[])
            n49 = for {
              tunnel: w87 -> [w100] mode=indexing
              tunnel: w70 -> [w99]
              n50 = property class="Arr (strict)"(reference=w100, "Number of Rows"=w99) -> ()  [unwired: 1 in, 2 out]
            }
            n51 = for {
              tunnel: w75 -> [w98] mode=indexing
              tunnel: w70 -> [w97]
              n52 = property class="Arr (strict)"(reference=w98, "Number of Rows"=w97) -> ()  [unwired: 1 in, 2 out]
            }
            n53 = property class="Arr (strict)"(reference=w86, "Number of Rows"=w70) -> ()  [unwired: 1 in, 2 out]
            n54 = property class="Arr (strict)"(reference=w71, "Number of Rows"=w70) -> ()  [unwired: 1 in, 2 out]
            n55 = property on="Camera Ready" class="Bool (strict)"(error in=w82, "Value"=w81) -> (error out=w69:errorcluster)  [unwired: 1 in, 1 out]
            n56 = shared-variable "NI-cRIO-9063-01c84dbf\\multiFunc-Lib.lvlib\\rt_app_status"(error in=w69) -> (w68:bool, error out=w65:errorcluster)
            n57 = property on="cRIO Ready" class="Bool (strict)"("Value"=w68) -> ()  [unwired: 2 in, 2 out]
            n58 = shared-variable "NI-cRIO-9063-01c84dbf\\multiFunc-Lib.lvlib\\get_loop_time"(error in=w65) -> (→"get_loop_time":u32, error out=w63:errorcluster)
            n59 = case shown="No Error" w63 {
              selector: w63 -> [w93 w95]
              tunnel: [rydberg_state_machine_states."Idle" rydberg_state_machine_states."Shutdown"] -> w67
              tunnel: [w93 w95] -> w66
              frame No Error {
              }
              frame Error {
              }
            }
          }
          event "Program Agilent": Value Change {
            n60 = event-data() -> ("NewVal"=w107:bool)  [unwired: 1 in, 5 out]
            n61 = Unbundle By Name(w106) -> ("Agilent E3631A Settings"=w102:T43)
            n62 = control-ref of="Agilent E3631A Settings"() -> (w101:refnum<vi>)
            n63 = case shown="True" w107 {
              tunnel: w102 -> [_ w115]
              tunnel: w105 -> [w108 w114]
              tunnel: [w108 w111] -> w104
              tunnel: w101 -> [_ w109]
              frame False {
              }
              frame True {
                n64 = call <vilib>:"Set Busy.vi"("error in (no error)"=w114, "disable click? (T)"=FALSE) -> ("error out"=w113:errorcluster)  [unwired: 8 in, 1 out]
                n65 = call "Neutral_Agilent_E3631A_20151027.vi"("error in (no error)"=w113, "Agilent E3631A RefNum"=w109, "Agilent E3631A Settings"=w115) -> ("error out"=w112:errorcluster)  [unwired: 8 in]
                n66 = call <vilib>:"Unset Busy.vi"("error in (no error)"=w112) -> ("error out"=w111:errorcluster)  [unwired: 10 in]
              }
            }
          }
          event "Update FPGA Ctrl": Value Change {
            n67 = event-data() -> ("NewVal"=w116:bool)  [unwired: 1 in, 5 out]
            n68 = case shown="True" w116 {
              tunnel: w119 -> [w120 w128]
              tunnel: [w120 w124] -> w118
              frame False {
              }
              frame True {
                # "Time delay so the user sees their button press"
                # "If an update was sent to the FPGA using \"Local\" mode on RT, then need to refresh the net_op_ctrl on this front panel"
                n69 = shared-variable "NI-cRIO-9063-01c84dbf\\multiFunc-Lib.lvlib\\net_op_ctrl"(error in=w128) -> (w127:T30, error out=w126:errorcluster)
                n70 = property on="FPGA_cntrl" class="Clust (strict)"(error in=w126, "Value"=w127) -> (error out=w122:errorcluster)  [unwired: 1 in, 1 out]
                n71 = call "Time Delay"("error in (no error)"=w122, "Delay Time (s)"=0.1) -> ("error out"=w121:errorcluster)  [unwired: 9 in]
                n72 = property on="Update FPGA Ctrl" class="Bool (strict)"(error in=w121, "Value"=FALSE ("Update FPGA Ctrl")) -> (error out=w124:errorcluster)  [unwired: 1 in, 1 out]
              }
            }
          }
          event "Intitialize PicoScope": Value Change {
            # "Another method to initialize Picoscope if it was not setup when neuKLEIN was started"
            n73 = event-data() -> ("NewVal"=w132:bool)  [unwired: 1 in, 5 out]
            n74 = property on="Picoscope Ready" class="Bool (strict)"() -> ("Value"=w129:bool)  [unwired: 2 in, 2 out]
            n75 = Unbundle By Name(w137) -> ("PicoScope"=w136:T39)
            n76 = Not(x=w129) -> (.not. x?=w131:bool)
            n77 = And(x=w131, y=w132) -> (x .and. y?=w130:bool)
            n78 = case shown="True" w130 {
              tunnel: w136 -> [_ w142]
              tunnel: w135 -> [w138 w147]
              tunnel: [w138 w146] -> w134